vi "Dresden R2R Sputter 03.02.2018 IY24.vi"() -> ()   [LabVIEW 2009] (continued)
                                }
                                frame #7 {
                                n27949 = Wait (ms)(milliseconds to wait=u32 100) -> ()  [unwired: 1 out]
                                n27950 = local write "Parameters_auto_set"(TRUE ("Parameters_auto_set")) -> ()
                                }
                                frame #8 {
                                n27951 = while {
                                i -> [w33022]
                                stop <- w33018 stop-if-true
                                n27952 = Wait Until Next ms Multiple(millisecond multiple=u32 300) -> ()  [unwired: 1 out]
                                n27953 = Greater?(x=w33022, y=100) -> (0:w33019:bool)
                                n27954 = local read "Parameters_auto_set"() -> (w33023:bool)
                                n27955 = case shown="False" w33023 {
                                tunnel: [TRUE FALSE] -> w33020
                                frame #0 {
                                }
                                frame #1 {
                                }
                                }
                                n27956 = Or(x=w33020, y=w33019) -> (x .or. y?=w33018:bool)
                                }
                                }
                                frame #9 {
                                n27957 = local read "R Tension Value"() -> (w33027:dbl)
                                n27958 = Wait (ms)(milliseconds to wait=u32 200) -> ()  [unwired: 1 out]
                                n27959 = local write "TC2_set_value"(w33027) -> ()
                                }
                                frame #10 {
                                n27960 = local write "TC2_auto_set"(TRUE ("TC1_auto_set")) -> ()
                                }
                                frame #11 {
                                w33030 = u16 2 items=["1", "2", "3", "4"] ("Target Chamber Sensor")
                                n27961 = local write "Target Chamber Sensor"(w33030) -> ()
                                }
                                frame #12 {
                                n27962 = local read "Total length"() -> (w33031:dbl)
                                n27963 = local write "Region"(w33031) -> ()
                                }
                                frame #13 {
                                n27964 = local read "Semi"() -> (w33032:bool)
                                n27965 = case shown="False" w33032 {
                                frame #0 {
                                n27966 = local write "Start_roll"(TRUE ("Start_roll")) -> ()
                                n27967 = Wait (ms)(milliseconds to wait=u32 300) -> ()  [unwired: 1 out]
                                }
                                frame #1 {
                                }
                                }
                                }
                                frame #14 {
                                n27968 = local read "Semi"() -> (w33035:bool)
                                n27969 = case shown="False" w33035 {
                                frame #0 {
                                n27970 = while {
                                stop <- w33039 stop-if-true
                                n27971 = Wait Until Next ms Multiple(millisecond multiple=u32 200 ("milliseconds to wait")) -> ()  [unwired: 1 out]
                                n27972 = local read "Start_roll"() -> (w33037:bool)
                                n27973 = Not(x=w33037) -> (.not. x?=w33036:bool)
                                n27974 = local read "Semi"() -> (w33040:bool)
                                n27975 = Or(x=w33036, y=w33040) -> (x .or. y?=w33039:bool)
                                }
                                }
                                frame #1 {
                                }
                                }
                                }
                                }
                                }
                                frame #1 {
                                }
                                }
                                }
                                frame #1 {
                                n27976 = disable-structure shown="Disabled" {
                                frame #0 {
                                # "OTHER"
                                n27977 = local read "Semi"() -> (w33041:bool)
                                n27978 = case shown="False" w33041 {
                                frame #0 {
                                n27979 = stacked-sequence {
                                frame #0 {
                                n27980 = local read "Semi"() -> (w33042:bool)
                                n27981 = case shown="False" w33042 {
                                frame #0 {
                                n27982 = while {
                                i -> [w33048]
                                stop <- w33045 stop-if-true
                                n27983 = Greater?(x=w33048, y=50) -> (0:w33047:bool)
                                n27984 = case shown="True" w33047 {
                                frame #0 {
                                }
                                frame #1 {
                                n27985 = local write "Error Message"("" ("Error Message")) -> ()
                                n27986 = local write "Semi"(TRUE ("Semi")) -> ()
                                }
                                }
                                n27987 = local read "Casette_servo_start/stop_di"() -> (w33044:bool)
                                n27988 = case shown="False" w33044 {
                                tunnel: [FALSE TRUE] -> w33043
                                frame #0 {
                                n27989 = local write "Casette_servo_start/stop_do"(TRUE ("Casette_servo_left_direction_do")) -> ()
                                n27990 = Wait Until Next ms Multiple(millisecond multiple=u32 500) -> ()  [unwired: 1 out]
                                }
                                frame #1 {
                                }
                                }
                                n27991 = local read "Semi"() -> (w33046:bool)
                                n27992 = Or(x=w33043, y=w33046) -> (x .or. y?=w33045:bool)
                                }
                                }
                                frame #1 {
                                }
                                }
                                }
                                frame #1 {
                                n27993 = local read "Semi"() -> (w33056:bool)
                                n27994 = case shown="False" w33056 {
                                frame #0 {
                                n27995 = while {
                                i -> [w33062]
                                stop <- w33059 stop-if-true
                                n27996 = Greater?(x=w33062, y=50) -> (0:w33061:bool)
                                n27997 = case shown="True" w33061 {
                                frame #0 {
                                }
                                frame #1 {
                                n27998 = local write "Error Message"("" ("Error Message")) -> ()
                                n27999 = local write "Semi"(TRUE ("Semi")) -> ()
                                }
                                }
                                n28000 = local read "Casette_servo_left_direction_di"() -> (w33058:bool)
                                n28001 = case shown="False" w33058 {
                                tunnel: [FALSE TRUE] -> w33057
                                frame #0 {
                                n28002 = local write "Casette_servo_left_direction_do"(TRUE ("Casette_servo_left_direction_do")) -> ()
                                n28003 = Wait Until Next ms Multiple(millisecond multiple=u32 200) -> ()  [unwired: 1 out]
                                }
                                frame #1 {
                                }
                                }
                                n28004 = local read "Semi"() -> (w33060:bool)
                                n28005 = Or(x=w33057, y=w33060) -> (x .or. y?=w33059:bool)
                                }
                                }
                                frame #1 {
                                }
                                }
                                }
                                frame #2 {
                                # "casette motion"
                                n28006 = while {
                                i -> [w33072]
                                stop <- w33070 stop-if-true
                                n28007 = Greater?(x=w33072, y=200) -> (0:w33073:bool)
                                n28008 = case shown="True" w33073 {
                                frame #0 {
                                }
                                frame #1 {
                                n28009 = local write "Semi"(TRUE ("Semi")) -> ()
                                }
                                }
                                n28010 = local read "Counter_read_data"() -> (w33078:i16)
                                n28011 = Greater?(x=w33078, y=i16 0) -> (0:w33076:bool)
                                n28012 = case shown="True" w33076 {
                                tunnel: [TRUE TRUE] -> w33075
                                frame #0 {
                                }
                                frame #1 {
                                n28013 = local write "Casette_servo_start/stop_do"(FALSE ("Casette_servo_start/stop_do")) -> ()
                                n28014 = Wait Until Next ms Multiple(millisecond multiple=u32 200) -> ()  [unwired: 1 out]
                                }
                                }
                                n28015 = local read "Semi"() -> (w33074:bool)
                                n28016 = Or(x=w33075, y=w33074) -> (x .or. y?=w33070:bool)
                                }
                                }
                                frame #3 {
                                n28017 = local read "Semi"() -> (w33084:bool)
                                n28018 = case shown="False" w33084 {
                                frame #0 {
                                n28019 = while {
                                i -> [w33090]
                                stop <- w33087 stop-if-true
                                n28020 = Greater?(x=w33090, y=50) -> (0:w33089:bool)
                                n28021 = case shown="True" w33089 {
                                frame #0 {
                                }
                                frame #1 {
                                n28022 = local write "Error Message"("" ("Error Message")) -> ()
                                n28023 = local write "Semi"(TRUE ("Semi")) -> ()
                                }
                                }
                                n28024 = local read "Casette_servo_start/stop_di"() -> (w33086:bool)
                                n28025 = case shown="True" w33086 {
                                tunnel: [TRUE FALSE] -> w33085
                                frame #0 {
                                }
                                frame #1 {
                                n28026 = local write "Casette_servo_start/stop_do"(FALSE ("Casette_servo_left_direction_do")) -> ()
                                n28027 = Wait Until Next ms Multiple(millisecond multiple=u32 500) -> ()  [unwired: 1 out]
                                }
                                }
                                n28028 = local read "Semi"() -> (w33088:bool)
                                n28029 = Or(x=w33085, y=w33088) -> (x .or. y?=w33087:bool)
                                }
                                }
                                frame #1 {
                                }
                                }
                                }
                                frame #4 {
                                n28030 = local read "Semi"() -> (w33098:bool)
                                n28031 = case shown="False" w33098 {
                                frame #0 {
                                n28032 = Wait Until Next ms Multiple(millisecond multiple=u32 5000 ("millisecond multiple 5")) -> ()  [unwired: 1 out]
                                }
                                frame #1 {
                                }
                                }
                                }
                                frame #5 {
                                n28033 = local read "Semi"() -> (w33100:bool)
                                n28034 = case shown="False" w33100 {
                                frame #0 {
                                n28035 = while {
                                i -> [w33106]
                                stop <- w33103 stop-if-true
                                n28036 = Greater?(x=w33106, y=50) -> (0:w33105:bool)
                                n28037 = case shown="True" w33105 {
                                frame #0 {
                                }
                                frame #1 {
                                n28038 = local write "Error Message"("" ("Error Message")) -> ()
                                n28039 = local write "Semi"(TRUE ("Semi")) -> ()
                                }
                                }
                                n28040 = local read "Casette_servo_start/stop_di"() -> (w33102:bool)
                                n28041 = case shown="False" w33102 {
                                tunnel: [FALSE TRUE] -> w33101
                                frame #0 {
                                n28042 = local write "Casette_servo_start/stop_do"(TRUE ("Casette_servo_left_direction_do")) -> ()
                                n28043 = Wait Until Next ms Multiple(millisecond multiple=u32 500) -> ()  [unwired: 1 out]
                                }
                                frame #1 {
                                }
                                }
                                n28044 = local read "Semi"() -> (w33104:bool)
                                n28045 = Or(x=w33101, y=w33104) -> (x .or. y?=w33103:bool)
                                }
                                }
                                frame #1 {
                                }
                                }
                                }
                                frame #6 {
                                n28046 = local read "Semi"() -> (w33114:bool)
                                n28047 = case shown="False" w33114 {
                                frame #0 {
                                n28048 = while {
                                i -> [w33120]
                                stop <- w33117 stop-if-true
                                n28049 = Greater?(x=w33120, y=50) -> (0:w33119:bool)
                                n28050 = case shown="True" w33119 {
                                frame #0 {
                                }
                                frame #1 {
                                n28051 = local write "Error Message"("" ("Error Message")) -> ()
                                n28052 = local write "Semi"(TRUE ("Semi")) -> ()
                                }
                                }
                                n28053 = local read "Casette_servo_left_direction_di"() -> (w33116:bool)
                                n28054 = case shown="True" w33116 {
                                tunnel: [TRUE FALSE] -> w33115
                                frame #0 {
                                }
                                frame #1 {
                                n28055 = local write "Casette_servo_left_direction_do"(FALSE ("Casette_servo_left_direction_do")) -> ()
                                n28056 = Wait Until Next ms Multiple(millisecond multiple=u32 200) -> ()  [unwired: 1 out]
                                }
                                }
                                n28057 = local read "Semi"() -> (w33118:bool)
                                n28058 = Or(x=w33115, y=w33118) -> (x .or. y?=w33117:bool)
                                }
                                }
                                frame #1 {
                                }
                                }
                                }
                                frame #7 {
                                # "casette motion"
                                n28059 = while {
                                i -> [w33131]
                                stop <- w33128 stop-if-true
                                n28060 = Greater?(x=w33131, y=200) -> (0:w33132:bool)
                                n28061 = case shown="True" w33132 {
                                frame #0 {
                                }
                                frame #1 {
                                n28062 = local write "Semi"(TRUE ("Semi")) -> ()
                                }
                                }
                                n28063 = local read "Counter_read_data"() -> (w33136:i16)
                                n28064 = Less?(x=w33136, y=i16 0) -> (x < y?=w33135:bool)
                                n28065 = case shown="True" w33135 {
                                tunnel: [TRUE TRUE] -> w33134
                                frame #0 {
                                }
                                frame #1 {
                                n28066 = local write "Casette_servo_start/stop_do"(FALSE ("Casette_servo_start/stop_do")) -> ()
                                n28067 = Wait Until Next ms Multiple(millisecond multiple=u32 200) -> ()  [unwired: 1 out]
                                }
                                }
                                n28068 = local read "Semi"() -> (w33133:bool)
                                n28069 = Or(x=w33134, y=w33133) -> (x .or. y?=w33128:bool)
                                }
                                }
                                frame #8 {
                                n28070 = local read "Semi"() -> (w33142:bool)
                                n28071 = case shown="False" w33142 {
                                frame #0 {
                                n28072 = while {
                                i -> [w33148]
                                stop <- w33145 stop-if-true
                                n28073 = Greater?(x=w33148, y=50) -> (0:w33147:bool)
                                n28074 = case shown="True" w33147 {
                                frame #0 {
                                }
                                frame #1 {
                                n28075 = local write "Error Message"("" ("Error Message")) -> ()
                                n28076 = local write "Semi"(TRUE ("Semi")) -> ()
                                }
                                }
                                n28077 = local read "Casette_servo_start/stop_di"() -> (w33144:bool)
                                n28078 = case shown="True" w33144 {
                                tunnel: [TRUE FALSE] -> w33143
                                frame #0 {
                                }
                                frame #1 {
                                n28079 = local write "Casette_servo_start/stop_do"(FALSE ("Casette_servo_left_direction_do")) -> ()
                                n28080 = Wait Until Next ms Multiple(millisecond multiple=u32 500) -> ()  [unwired: 1 out]
                                }
                                }
                                n28081 = local read "Semi"() -> (w33146:bool)
                                n28082 = Or(x=w33143, y=w33146) -> (x .or. y?=w33145:bool)
                                }
                                }
                                frame #1 {
                                }
                                }
                                }
                                frame #9 {
                                n28083 = local read "Semi"() -> (w33156:bool)
                                n28084 = case shown="False" w33156 {
                                frame #0 {
                                }
                                frame #1 {
                                }
                                }
                                }
                                }
                                }
                                frame #1 {
                                }
                                }
                                }
                                frame #1 {
                                }
                                }
                                }
                                }
                                }
                                frame #1 {
                                }
                                }
                                }
                                frame #1 {
                                n28085 = local read "Semi"() -> (w33157:bool)
                                n28086 = case shown="False" w33157 {
                                frame #0 {
                                n28087 = Wait (ms)(milliseconds to wait=u32 1000) -> ()  [unwired: 1 out]
                                n28088 = local write "SDC1 29"(TRUE ("SDC1 29")) -> ()
                                }
                                frame #1 {
                                }
                                }
                                }
                                }
                                }
                                frame #27 {
                                n28089 = local read "Semi"() -> (w33160:bool)
                                n28090 = case shown="False" w33160 {
                                frame #0 {
                                n28091 = Wait (ms)(milliseconds to wait=u32 2500) -> ()  [unwired: 1 out]
                                n28092 = local write "Cnt_Do_Buzzer"(TRUE ("SDC1 30")) -> ()
                                n28093 = local write "SDC1 30"(TRUE ("SDC1 30")) -> ()
                                }
                                frame #1 {
                                }
                                }
                                }
                                frame #28 {
                                n28094 = local read "Semi"() -> (w33164:bool)
                                n28095 = case shown="False" w33164 {
                                frame #0 {
                                n28096 = Wait (ms)(milliseconds to wait=u32 1000) -> ()  [unwired: 1 out]
                                n28097 = local write "Cnt_Do_Buzzer"(FALSE ("SDC1 30")) -> ()
                                }
                                frame #1 {
                                }
                                }
                                }
                                }
                                }
                                frame #1 {
                                }
                                }
                                }
                              }
                            }
                          }
                        }
                        frame #2 {
                          n28098 = local read "MW_RF_Interlock"() -> (w33167:dbl)
                          n28099 = local read "Ch4_pressure2"() -> (w33171:dbl)
                          n28100 = local read "started_up_ch4"() -> (w33169:bool)
                          n28101 = In Range and Coerce(upper limit=w33167, x=w33171, lower limit=1e-08) -> (In Range?=w33172:bool)  [unwired: 1 out]
                          n28102 = And(x=w33172, y=w33169) -> (x .and. y?=w33168:bool)
                          n28103 = case shown="True" w33168 {
                            frame #0 {
                            }
                            frame #1 {
                              n28104 = local read "Semi"() -> (w33173:bool)
                              n28105 = case shown="False" w33173 {
                                frame #0 {
                                n28106 = stacked-sequence {
                                frame #0 {
                                n28107 = stacked-sequence {
                                frame #0 {
                                n28108 = local read "Semi"() -> (w33174:bool)
                                n28109 = case shown="False" w33174 {
                                frame #0 {
                                w33177 = FALSE ("Casette_servo_start/stop_do")
                                n28110 = local write "Ch4_Sov_Ar_do"(FALSE ("Ch1_Sov_Ar_do")) -> ()
                                n28111 = local write "RF_host_auto"(TRUE ("Dc_host_auto")) -> ()
                                n28112 = local write "Ar_auto_set_zero_ch4"(TRUE ("Dc_auto_set_zero")) -> ()
                                n28113 = local write "final_process_messages"("Coating was Completed" ("final_process_messages")) -> ()
                                n28114 = local write "system_status"("Coating Mode is Active" ("system_status")) -> ()
                                n28115 = local write "Casette_servo_start/stop_do"(w33177) -> ()
                                n28116 = local write "Tension_controllers_start/stop_do"(w33177) -> ()
                                }
                                frame #1 {
                                }
                                }
                                }
                                frame #1 {
                                n28117 = local read "Semi"() -> (w33181:bool)
                                n28118 = case shown="False" w33181 {
                                frame #0 {
                                n28119 = Wait (ms)(milliseconds to wait=u32 2500) -> ()  [unwired: 1 out]
                                }
                                frame #1 {
                                }
                                }
                                }
                                frame #2 {
                                n28120 = local read "Semi"() -> (w33183:bool)
                                n28121 = case shown="False" w33183 {
                                frame #0 {
                                n28122 = local write "Ch4_SRV_start_stop_do"(FALSE ("Ch1_SRV_start_stop_do")) -> ()
                                }
                                frame #1 {
                                }
                                }
                                }
                                frame #3 {
                                n28123 = local read "Semi"() -> (w33185:bool)
                                n28124 = case shown="False" w33185 {
                                frame #0 {
                                n28125 = Wait (ms)(milliseconds to wait=u32 2500) -> ()  [unwired: 1 out]
                                }
                                frame #1 {
                                }
                                }
                                }
                                frame #4 {
                                n28126 = local read "Semi"() -> (w33187:bool)
                                n28127 = case shown="False" w33187 {
                                frame #0 {
                                n28128 = Wait (ms)(milliseconds to wait=u32 1000) -> ()  [unwired: 1 out]
                                n28129 = local write "SDC1 1"(TRUE ("CMW1")) -> ()
                                }
                                frame #1 {
                                }
                                }
                                }
                                }
                                }
                                frame #1 {
                                n28130 = local read "ch_present_position"() -> (w33192:dbl)
                                n28131 = Not Equal?(x=w33192, y=4.0) -> (x != y?=w33190:bool)
                                n28132 = case shown="True" w33190 {
                                frame #0 {
                                }
                                frame #1 {
                                n28133 = stacked-sequence {
                                frame #0 {
                                n28134 = local write "Set chamber"(4.0 ("Set chamber")) -> ()
                                n28135 = Wait (ms)(milliseconds to wait=u32 100) -> ()  [unwired: 1 out]
                                }
                                frame #1 {
                                n28136 = local write "Auto_set_transfer"(TRUE ("Auto_set_transfer")) -> ()
                                }
                                frame #2 {
                                n28137 = while {
                                stop <- w33197 stop-if-true
                                n28138 = Wait Until Next ms Multiple(millisecond multiple=u32 300) -> ()  [unwired: 1 out]
                                n28139 = local read "Auto_set_transfer"() -> (w33198:bool)
                                n28140 = local read "Semi"() -> (w33200:bool)
                                n28141 = Not(x=w33198) -> (.not. x?=w33199:bool)
                                n28142 = Or(x=w33199, y=w33200) -> (x .or. y?=w33197:bool)
                                }
                                }
                                frame #3 {
                                n28143 = Wait (ms)(milliseconds to wait=u32 300) -> ()  [unwired: 1 out]
                                n28144 = local write "SRF 15"(TRUE ("SMW1 2")) -> ()
                                }
                                }
                                }
                                }
                                }
                                frame #2 {
                                # "WATER FLOW CONTROL OPEN"
                                n28145 = stacked-sequence {
                                frame #0 {
                                n28146 = local read "Semi"() -> (w33203:bool)
                                n28147 = case shown="False" w33203 {
                                frame #0 {
                                n28148 = while {
                                i -> [w33209]
                                stop <- w33204 stop-if-true
                                n28149 = Greater?(x=w33209, y=100) -> (0:w33208:bool)
                                n28150 = case shown="True" w33208 {
                                frame #0 {
                                }
                                frame #1 {
                                n28151 = local write "Semi"(TRUE ("Semi")) -> ()
                                n28152 = local write "Error Message"("Coating Process  \nwas cancelled.\nPlease check water \nflow connection." ("Error Message")) -> ()
                                }
                                }
                                n28153 = local read "Ch3_WFS_di"() -> (w33207:bool)
                                n28154 = case shown="True" w33207 {
                                tunnel: [TRUE FALSE] -> w33206
                                frame #0 {
                                }
                                frame #1 {
                                n28155 = local write "Ch3_WFC_do"(FALSE ("Ch1_WFC_do")) -> ()
                                n28156 = Wait Until Next ms Multiple(millisecond multiple=u32 200) -> ()  [unwired: 1 out]
                                }
                                }
                                n28157 = local read "Semi"() -> (w33205:bool)
                                n28158 = Or(x=w33206, y=w33205) -> (x .or. y?=w33204:bool)
                                }
                                }
                                frame #1 {
                                }
                                }
                                }
                                frame #1 {
                                n28159 = local read "Semi"() -> (w33217:bool)
                                n28160 = case shown="False" w33217 {
                                frame #0 {
                                n28161 = while {
                                i -> [w33223]
                                stop <- w33218 stop-if-true
                                n28162 = Greater?(x=w33223, y=100) -> (0:w33222:bool)
                                n28163 = case shown="True" w33222 {
                                frame #0 {
                                }
                                frame #1 {
                                n28164 = local write "Semi"(TRUE ("Semi")) -> ()
                                n28165 = local write "Error Message"("Coating Process  \nwas cancelled.\nPlease check water \nflow connection." ("Error Message")) -> ()
                                }
                                }
                                n28166 = local read "Ch1_WFS_di"() -> (w33221:bool)
                                n28167 = case shown="True" w33221 {
                                tunnel: [TRUE FALSE] -> w33220
                                frame #0 {
                                }
                                frame #1 {
                                n28168 = local write "Ch1_WFC_do"(FALSE ("Ch1_WFC_do")) -> ()
                                n28169 = Wait Until Next ms Multiple(millisecond multiple=u32 200) -> ()  [unwired: 1 out]
                                }
                                }
                                n28170 = local read "Semi"() -> (w33219:bool)
                                n28171 = Or(x=w33220, y=w33219) -> (x .or. y?=w33218:bool)
                                }
                                }
                                frame #1 {
                                }
                                }
                                }
                                frame #2 {
                                n28172 = local read "Semi"() -> (w33231:bool)
                                n28173 = case shown="False" w33231 {
                                frame #0 {
                                n28174 = while {
                                i -> [w33237]
                                stop <- w33232 stop-if-true
                                n28175 = Greater?(x=w33237, y=100) -> (0:w33236:bool)
                                n28176 = case shown="True" w33236 {
                                frame #0 {
                                }
                                frame #1 {
                                n28177 = local write "Semi"(TRUE ("Semi")) -> ()
                                n28178 = local write "Error Message"("Coating Process  \nwas cancelled.\nPlease check water \nflow connection." ("Error Message")) -> ()
                                }
                                }
                                n28179 = local read "Ch2_WFS_di"() -> (w33235:bool)
                                n28180 = case shown="True" w33235 {
                                tunnel: [TRUE FALSE] -> w33234
                                frame #0 {
                                }
                                frame #1 {
                                n28181 = local write "Ch2_WFC_do"(FALSE ("Ch1_WFC_do")) -> ()
                                n28182 = Wait Until Next ms Multiple(millisecond multiple=u32 200) -> ()  [unwired: 1 out]
                                }
                                }
                                n28183 = local read "Semi"() -> (w33233:bool)
                                n28184 = Or(x=w33234, y=w33233) -> (x .or. y?=w33232:bool)
                                }
                                }
                                frame #1 {
                                }
                                }
                                }
                                frame #3 {
                                n28185 = local read "Semi"() -> (w33245:bool)
                                n28186 = case shown="False" w33245 {
                                frame #0 {
                                n28187 = while {
                                i -> [w33251]
                                stop <- w33246 stop-if-true
                                n28188 = Greater?(x=w33251, y=100) -> (0:w33250:bool)
                                n28189 = case shown="True" w33250 {
                                frame #0 {
                                }
                                frame #1 {
                                n28190 = local write "Semi"(TRUE ("Semi")) -> ()
                                n28191 = local write "Error Message"("Coating Process  \nwas cancelled.\nPlease check water \nflow connection." ("Error Message")) -> ()
                                }
                                }
                                n28192 = local read "Ch4_WFS_di"() -> (w33249:bool)
                                n28193 = case shown="False" w33249 {
                                tunnel: [FALSE TRUE] -> w33248
                                frame #0 {
                                n28194 = local write "Ch4_WFC_do"(TRUE ("Ch1_WFC_do")) -> ()
                                n28195 = Wait Until Next ms Multiple(millisecond multiple=u32 200) -> ()  [unwired: 1 out]
                                }
                                frame #1 {
                                }
                                }
                                n28196 = local read "Semi"() -> (w33247:bool)
                                n28197 = Or(x=w33248, y=w33247) -> (x .or. y?=w33246:bool)
                                }
                                }
                                frame #1 {
                                }
                                }
                                }
                                frame #4 {
                                n28198 = local read "Semi"() -> (w33259:bool)
                                n28199 = case shown="False" w33259 {
                                frame #0 {
                                n28200 = local write "SDC1 2"(TRUE ("SDC1 2")) -> ()
                                n28201 = Wait (ms)(milliseconds to wait=u32 1000) -> ()  [unwired: 1 out]
                                }
                                frame #1 {
                                }
                                }
                                }
                                }
                                }
                                frame #3 {
                                # "BG-BV open"
                                n28202 = stacked-sequence {
                                frame #0 {
                                n28203 = local read "Semi"() -> (w33262:bool)
                                n28204 = case shown="False" w33262 {
                                frame #0 {
                                n28205 = while {
                                i -> [w33268]
                                stop <- w33263 stop-if-true
                                n28206 = Greater?(x=w33268, y=50) -> (0:w33267:bool)
                                n28207 = case shown="True" w33267 {
                                frame #0 {
                                }
                                frame #1 {
                                n28208 = local write "Semi"(TRUE ("Semi")) -> ()
                                n28209 = local write "Error Message"("Coating Process  \nwas cancelled.\nPlease check \nBG-BV connection." ("Error Message")) -> ()
                                }
                                }
                                n28210 = local read "Ch4_Bg_bv_di"() -> (w33266:bool)
                                n28211 = case shown="False" w33266 {
                                tunnel: [FALSE TRUE] -> w33265
                                frame #0 {
                                n28212 = local write "Ch4_Bg_bv_do"(TRUE ("Ch1_WFC_do")) -> ()
                                n28213 = Wait Until Next ms Multiple(millisecond multiple=u32 200) -> ()  [unwired: 1 out]
                                }
                                frame #1 {
                                }
                                }
                                n28214 = local read "Semi"() -> (w33264:bool)
                                n28215 = Or(x=w33265, y=w33264) -> (x .or. y?=w33263:bool)
                                }
                                }
                                frame #1 {
                                }
                                }
                                }
                                frame #1 {
                                n28216 = local read "Semi"() -> (w33276:bool)
                                n28217 = case shown="False" w33276 {
                                frame #0 {
                                n28218 = Wait (ms)(milliseconds to wait=u32 1000) -> ()  [unwired: 1 out]
                                n28219 = local write "SDC1 4"(TRUE ("SDC1 4")) -> ()
                                }
                                frame #1 {
                                }
                                }
                                }
                                }
                                }
                                frame #4 {
                                # "Baratron set zero"
                                n28220 = stacked-sequence {
                                frame #0 {
                                n28221 = local write "Pc_bv4_auto_baratron_set_zero"(TRUE ("Pc_bv2_auto_baratron_set_zero")) -> ()
                                }
                                frame #1 {
                                n28222 = while {
                                i -> [w33284]
                                stop <- w33281 stop-if-true
                                n28223 = Greater?(x=w33284, y=50 ("Baratron set zero time 2")) -> (0:w33283:bool)
                                n28224 = case shown="True" w33283 {
                                frame #0 {
                                }
                                frame #1 {
                                n28225 = local write "Semi"(TRUE ("Semi")) -> ()
                                n28226 = local write "Error Message"("" ("Error Message")) -> ()
                                }
                                }
                                n28227 = local read "Pressure 4"() -> (w33280:i32)
                                n28228 = Less?(x=w33280, y=0.1 ("Pressure Check for baratron set zero")) -> (x < y?=w33287:bool)
                                n28229 = case shown="False" w33287 {
                                tunnel: [FALSE TRUE] -> w33286
                                frame #0 {
                                n28230 = Wait Until Next ms Multiple(millisecond multiple=u32 200) -> ()  [unwired: 1 out]
                                }
                                frame #1 {
                                }
                                }
                                n28231 = local read "Semi"() -> (w33285:bool)
                                n28232 = Or(x=w33286, y=w33285) -> (x .or. y?=w33281:bool)
                                }
                                }
                                frame #2 {
                                n28233 = local read "Semi"() -> (w33294:bool)
                                n28234 = case shown="False" w33294 {
                                frame #0 {
                                n28235 = local write "SDC1 2b"(TRUE ("SDC1 2b")) -> ()
                                n28236 = Wait (ms)(milliseconds to wait=u32 1000) -> ()  [unwired: 1 out]
                                }
                                frame #1 {
                                }
                                }
                                }
                                }
                                }
                                frame #5 {
                                # "CC CLOSE"
                                n28237 = stacked-sequence {
                                frame #0 {
                                n28238 = local read "Semi"() -> (w33297:bool)
                                n28239 = case shown="False" w33297 {
                                frame #0 {
                                n28240 = while {
                                i -> [w33303]
                                stop <- w33298 stop-if-true
                                n28241 = Greater?(x=w33303, y=50) -> (0:w33302:bool)